vi "ContourPlot v4.6 IV.vi"() -> ()   [LabVIEW 2024]
uses:
  diff para.ctl
  graph para.ctl
  <vilib>/Analysis/NI_AALPro.lvlib
  <vilib>/gmath/NI_Gmath.lvlib
panel:
  out "Field data":dbl[](array[numeric])=[-8.0, -7.95, -7.9, -7.85, -7.8, -7.75, -7.7, -7.65, -7.6, -7.55, -7.5, -7.45, -7.4, -7.35, -7.3, -7.25, -7.2, -7.15, -7.1, -7.05, -7.0, -6.95, -6.9, -6.85, -6.8, -6.75, -6.7, -6.65, -6.6, -6.55, -6.5, -6.45, -6.4, -6.35, -6.3, -6.25, -6.2, -6.15, -6.1, -6.05, -6.0, -5.95, -5.9, -5.85, -5.8, -5.75, -5.7, -5.65, -5.6, -5.55, -5.5, -5.45, -5.4, -5.35, -5.3, -5.25, -5.2, -5.15, -5.1, -5.05, -5.0, -4.95, -4.9, -4.85, -4.8, -4.75, -4.7, -4.65, -4.6, -4.55, -4.5, -4.45, -4.4, -4.35, -4.3, -4.25, -4.2, -4.15, -4.1, -4.05, -4.0, -3.95, -3.9, -3.85, -3.8, -3.75, -3.7, -3.65, -3.6, -3.55, -3.5, -3.45, -3.4, -3.35, -3.3, -3.25, -3.2, -3.15, -3.1, -3.05, -3.0, -2.95, -2.9, -2.85, -2.8, -2.75, -2.7, -2.65, -2.6, -2.55, -2.5, -2.45, -2.4, -2.35, -2.3, -2.25, -2.2, -2.15, -2.1, -2.05, -2.0, -1.95, -1.9, -1.85, -1.8, -1.75, -1.7, -1.65, -1.6, -1.55, -1.5, -1.45, -1.4, -1.35, -1.3, -1.25, -1.2, -1.15, -1.1, -1.05, -1.0, -0.95, -0.9, -0.85, -0.8, -0.75, -0.7, -0.65, -0.6, -0.55, -0.5, -0.45, -0.4, -0.35, -0.3, -0.25, -0.2, -0.15, -0.1, -0.05, 0.0, 0.05, 0.1, 0.15, 0.2, 0.25, 0.3, 0.35, 0.4, 0.45, 0.5, 0.55, 0.6, 0.65, 0.7, 0.75, 0.8, 0.85, 0.9, 0.95, 1.0, 1.05, 1.1, 1.15, 1.2, 1.25, 1.3, 1.35, 1.4, 1.45, 1.5, 1.55, 1.6, 1.65, 1.7, 1.75, 1.8, 1.85, 1.9, 1.95, 2.0, 2.05, 2.1, 2.15, 2.2, 2.25, 2.3, 2.35, 2.4, 2.45, 2.5, 2.55, 2.6, 2.65, 2.7, 2.75, 2.8, 2.85, 2.9, 2.95, 3.0, 3.05, 3.1, 3.15, 3.2, 3.25, 3.3, 3.35, 3.4, 3.45, 3.5, 3.55, 3.6, 3.65, 3.7, 3.75, 3.8, 3.85, 3.9, 3.95, 4.0, 4.05, 4.1, 4.15, 4.2, 4.25, 4.3, 4.35, 4.4, 4.45, 4.5, 4.55, 4.6, 4.65, 4.7, 4.75, 4.8, 4.85, 4.9, 4.95, 5.0, 5.05, 5.1, 5.15, 5.2, 5.25, 5.3, 5.35, 5.4, 5.45, 5.5, 5.55, 5.6, 5.65, 5.7, 5.75, 5.8, 5.85, 5.9, 5.95, 6.0, 6.05, 6.1, 6.15, 6.2, 6.25, 6.3, 6.35, 6.4, 6.45, 6.5, 6.55, 6.6, 6.65, 6.7, 6.75, 6.8, 6.85, 6.9, 6.95, 7.0, 7.05, 7.1, 7.15, 7.2, 7.25, 7.3, 7.35, 7.4, 7.45, 7.5, 7.55, 7.6, 7.65, 7.7, 7.75, 7.8, 7.85, 7.9, 7.95, 8.0]
  in  "Help":bool caption="load data"
  out "smoothed dIV buffer":dbl[][](array[numeric])
  in  "diff para":T1={"x0"=-1.0, "Ic0"=2.0, "h0"=1.0, "y0"=0.0}
  in  "Plot reference":bool caption="load data"
  out "smoothed dIV":dbl[][](array[numeric])
  out "smoothed data":dbl[][](array[numeric])
  in  "smooth n":i32=10
  out "IVdata":dbl[][](array[numeric])
  in  "load data":bool
  out "Status":string="Stopped"
  in  "stop":bool
  in  "Begin":i32
  in  "length":i32=1000
  in  "Contact Resistance":dbl
  in  "Tab Control 2":enum32{"IV plots", "IV smoothed", "dV/dI"}(tab)
  in  "Method":string(combo)="Raw data"
  in  "extract contour":bool caption="load data"
  out "IV Intensity":dbl[][](graph)
  out "IV":T2(graph)
  in  "polynomial order":i32=22
  out "Contour":cluster{"Field data":dbl[], dbl[]}(graph)
  in  "Threshold":dbl
  out "dX/2":dbl=2.3584433814410506
  out "dX":dbl=4.716886762882101
  in  "Plot contour line":bool
  out "IV smoothed intensity":dbl[][](graph)
  out "Smooth IV":cluster{dbl[], "Intensity Graph":dbl[]}(graph)
  in  "Set diff parameter":bool caption="load data"
  out "dVdI Intensity":dbl[][](graph)
  out "dV/dI":cluster{dbl[], "Intensity Graph":dbl[]}(graph)
  in  "book number":i32=820
  in  "file path":path=path "C:/Users/gyue/Desktop/GA01_202401"
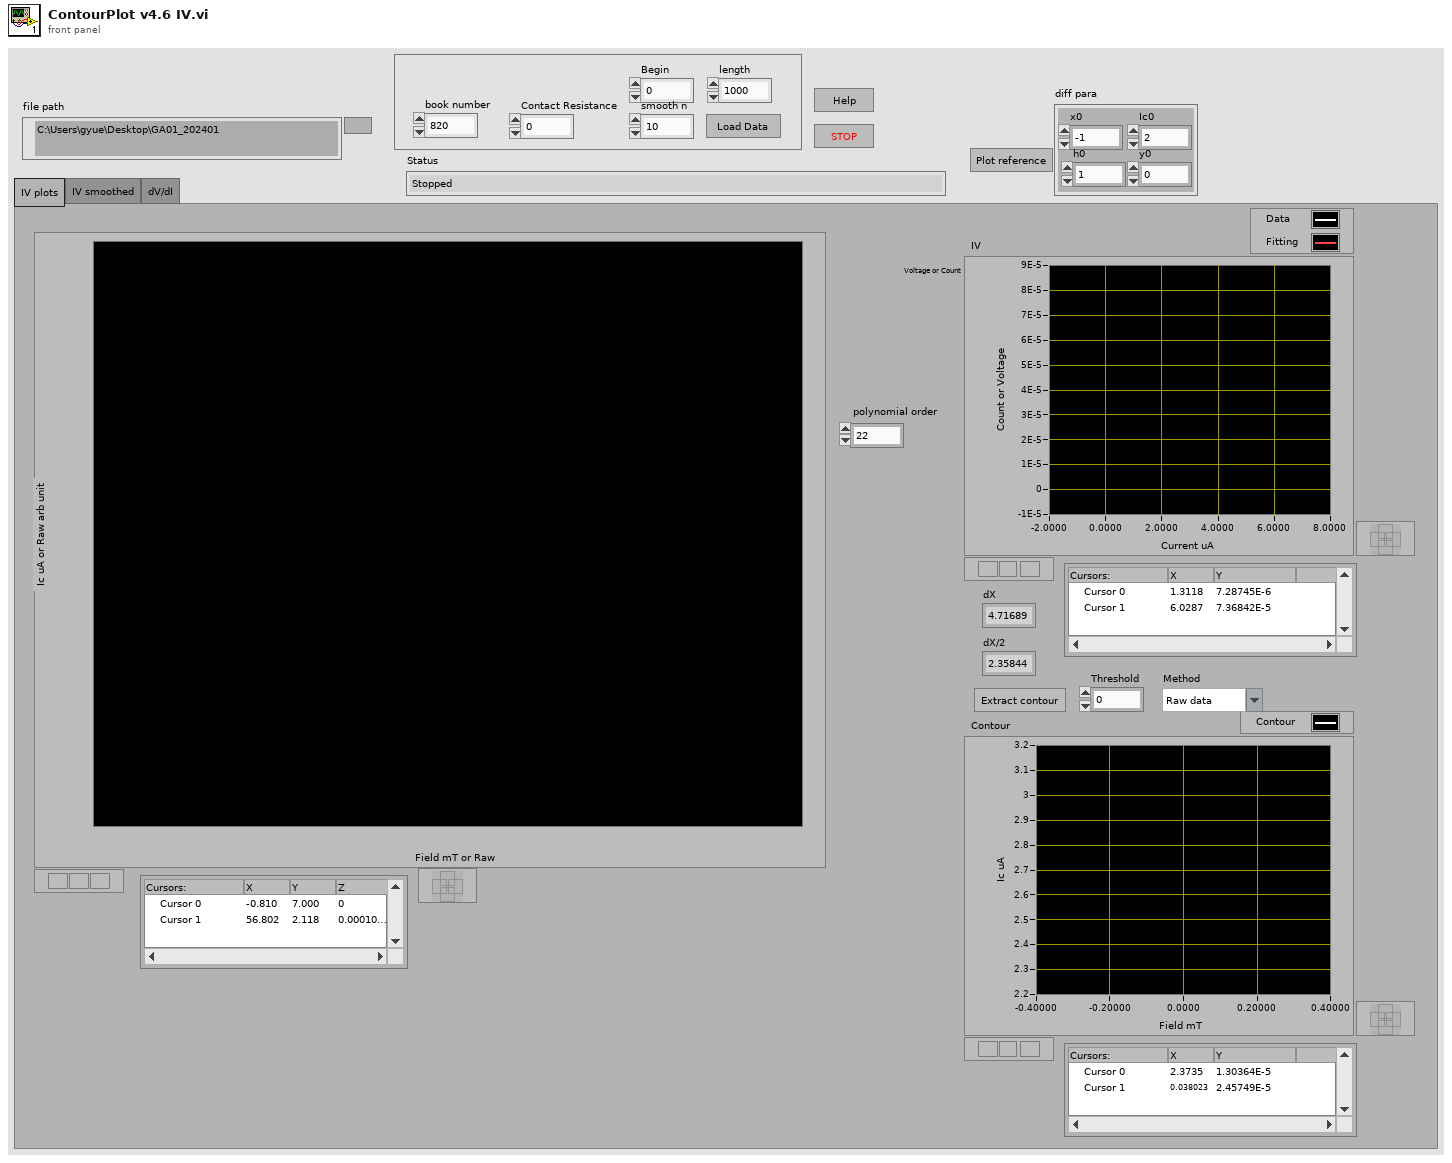
[diagram p1: front panel]
types:
  T1 = typedef "diff para.ctl" = cluster{"x0":dbl, "Ic0":dbl, "h0":dbl, "y0":dbl}
  T2 = cluster{"X":dbl[], "Best Polynomial Fit":dbl[]}[]
  T3 = typedef "graph para.ctl" = cluster{"x offset":dbl, "y offset":dbl, "x scale":dbl, "y scale":dbl}
  T4 = typedef "LVCursorListTypeDef.ctl" = cluster{"Name":string, "Color":u32, "Style":u8, "Point Style":u8, "Name Visible":bool, "Allow Drag":bool, "Cursor Mode":u32, "Plot":i32, "Index":i32, "Position":cluster{"X":dbl, "Y":dbl}, "X Scale":u32, "Y Scale":u32, "Watch Plots":i32[], "Watch All Plots":bool, "Plot Area":i32, "Label Offset":cluster{"X":dbl, "Y":dbl}}[]
  T5 = cluster{"Name":string, "Color":u32, "Style":u8, "Point Style":u8, "Name Visible":bool, "Allow Drag":bool, "Cursor Mode":u32, "Plot":i32, "Index":i32, "Position":cluster{"X":dbl, "Y":dbl}, "X Scale":u32, "Y Scale":u32, "Watch Plots":i32[], "Watch All Plots":bool, "Plot Area":i32, "Label Offset":cluster{"X":dbl, "Y":dbl}}
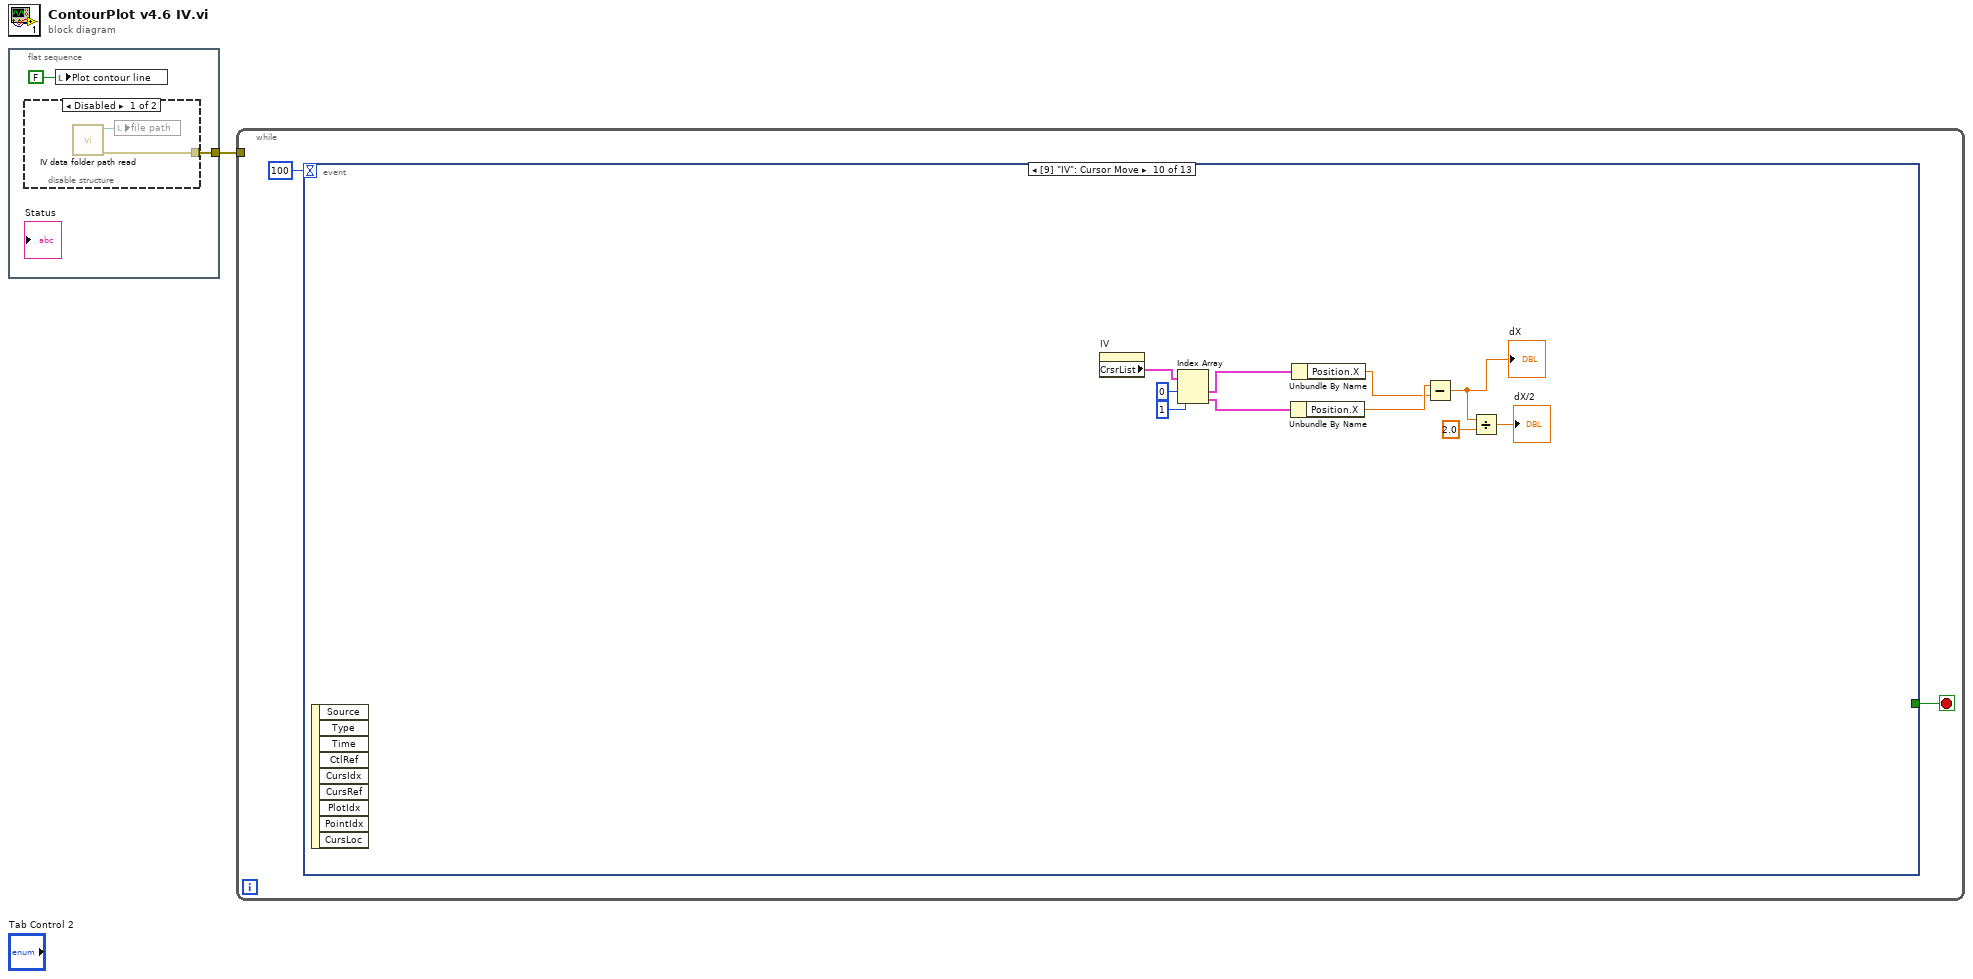
[diagram p0: block diagram]
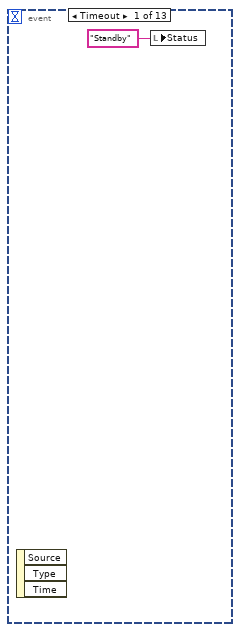
[diagram p3: hidden frame]
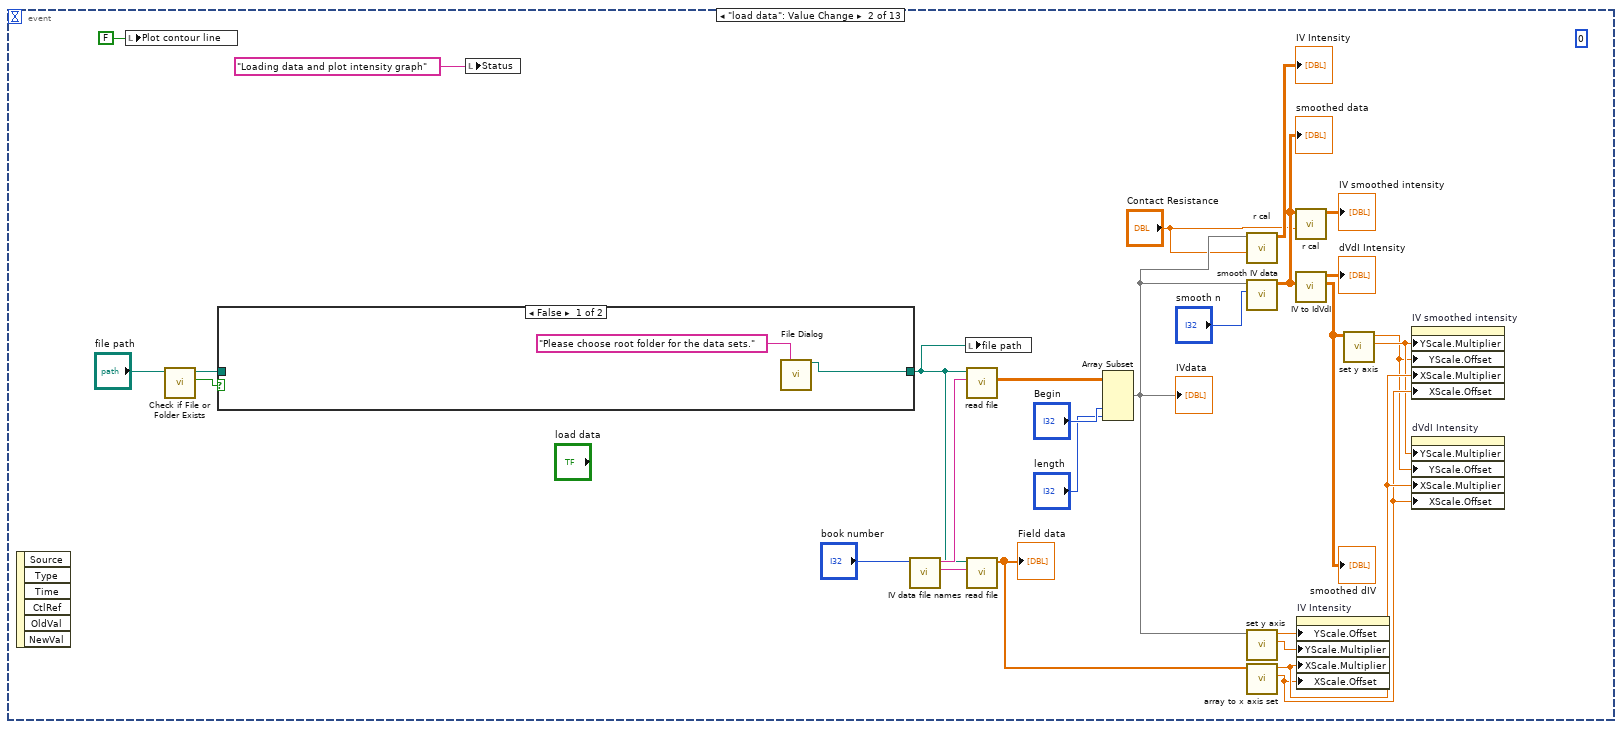
[diagram p4: hidden frame]
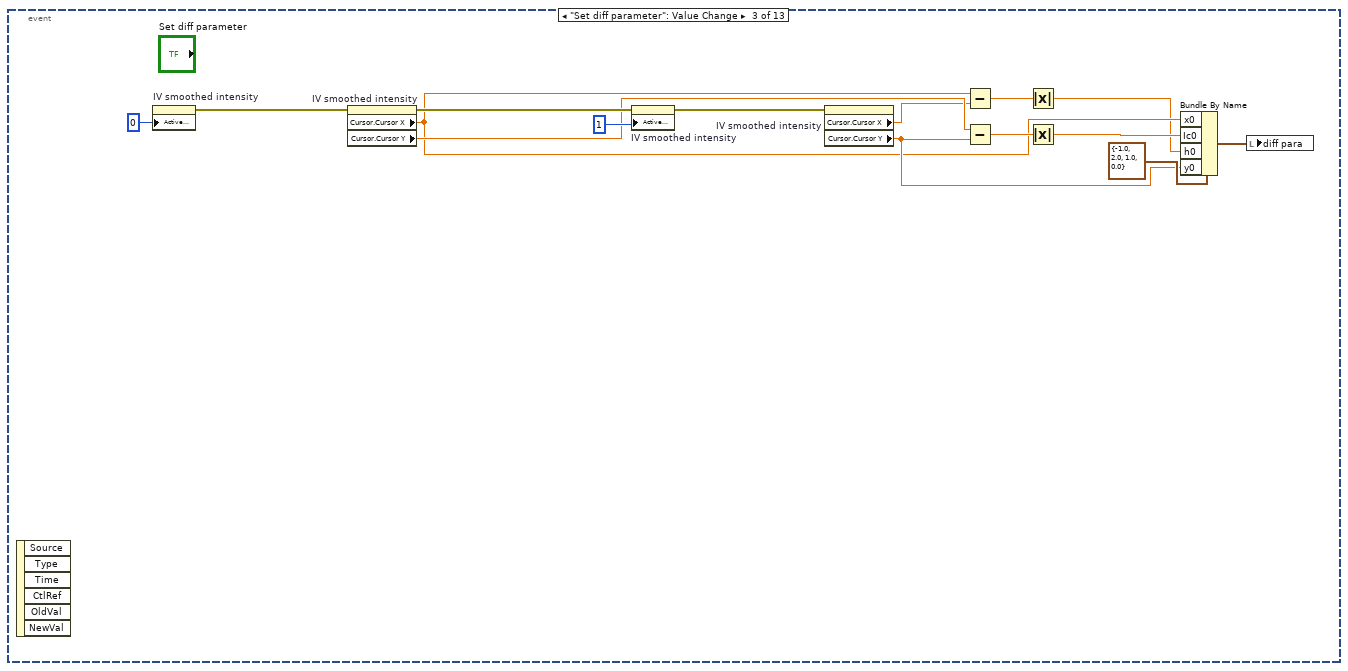
[diagram p6: hidden frame]
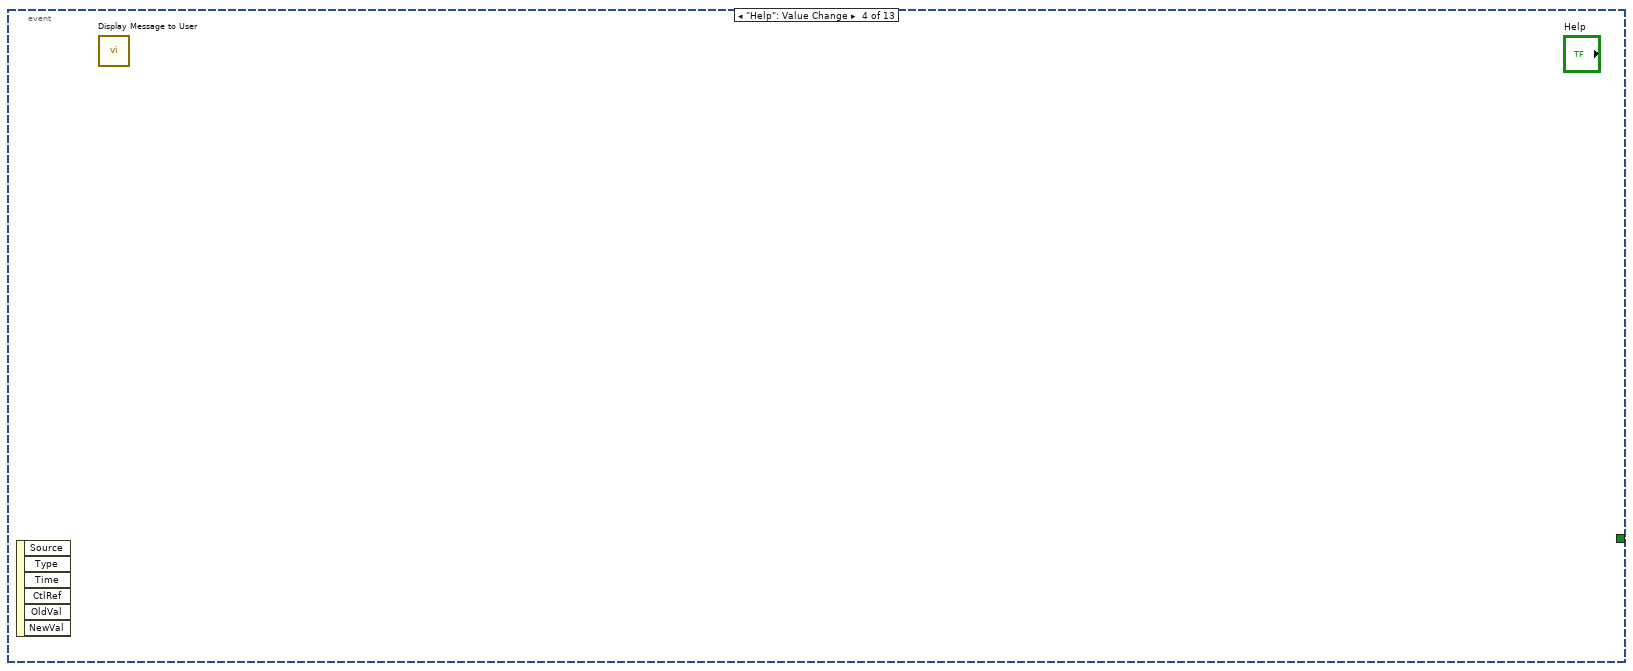
[diagram p7: hidden frame]
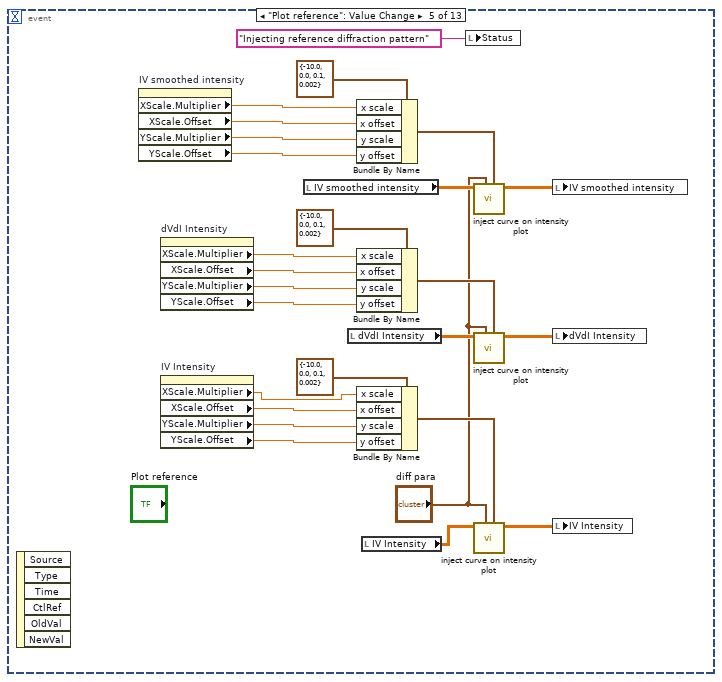
[diagram p8: hidden frame]
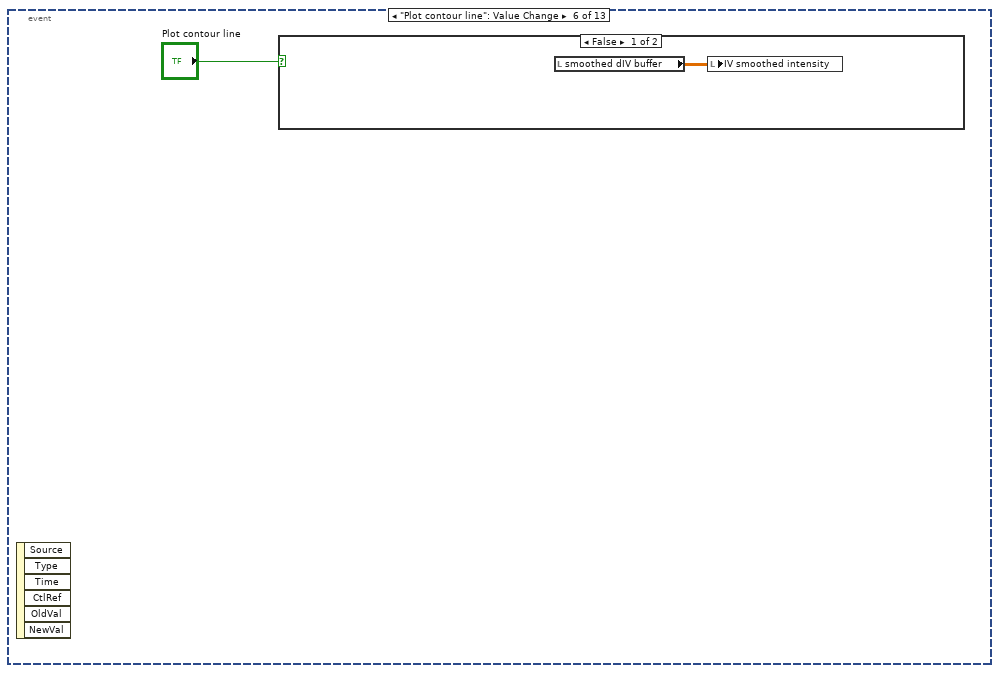
[diagram p9: hidden frame]
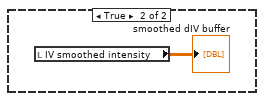
[diagram p10: hidden frame]
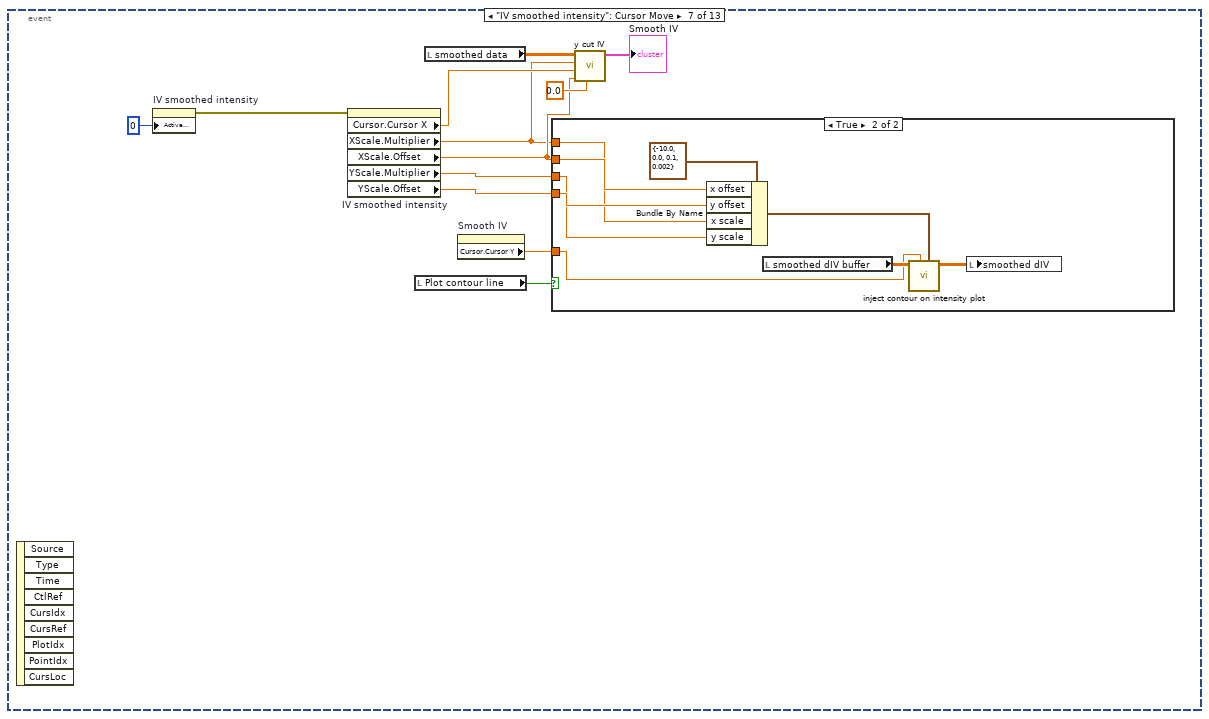
[diagram p11: hidden frame]
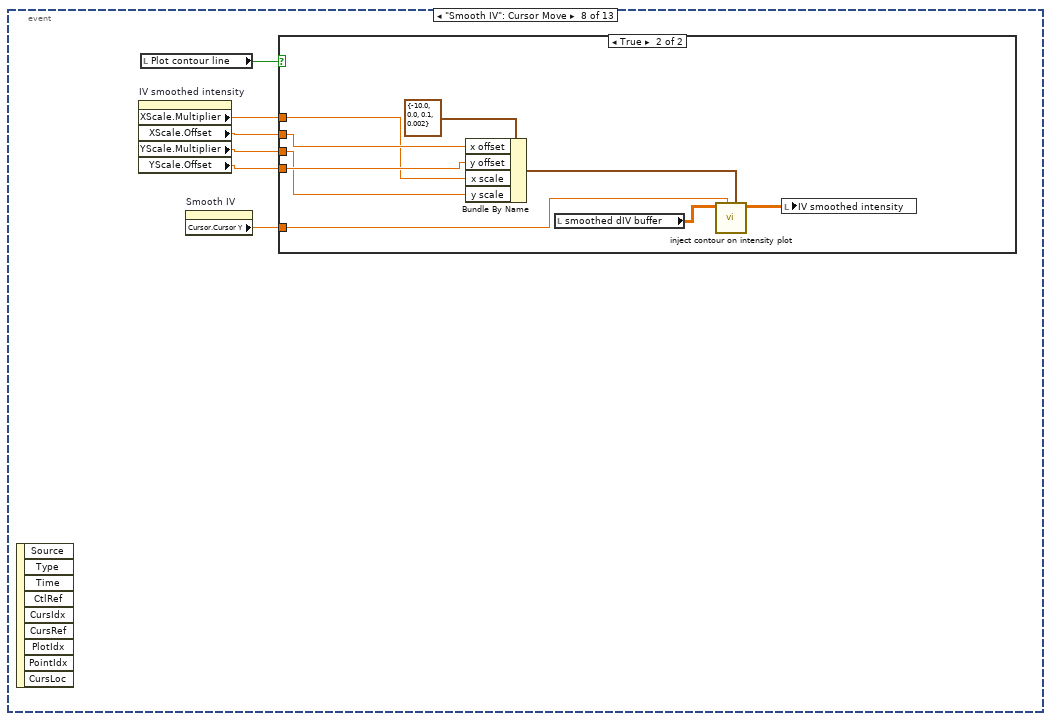
[diagram p13: hidden frame]
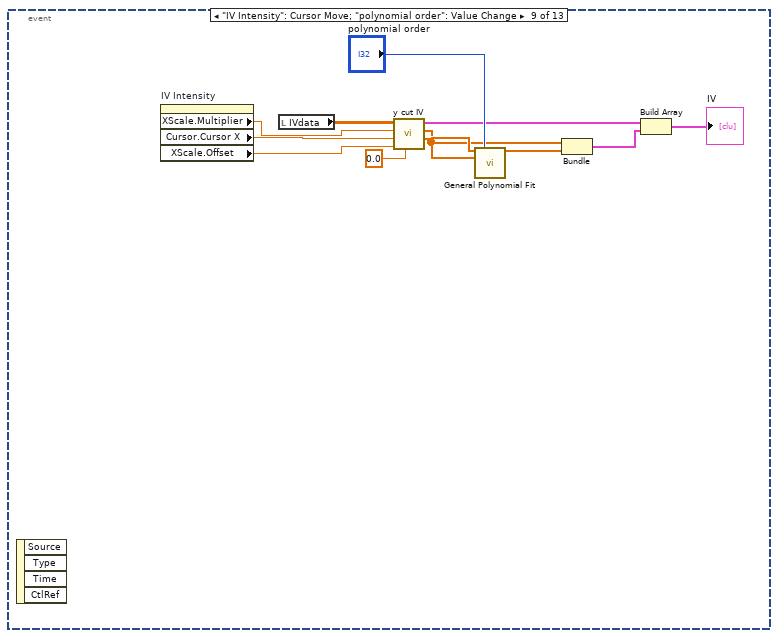
[diagram p15: hidden frame]
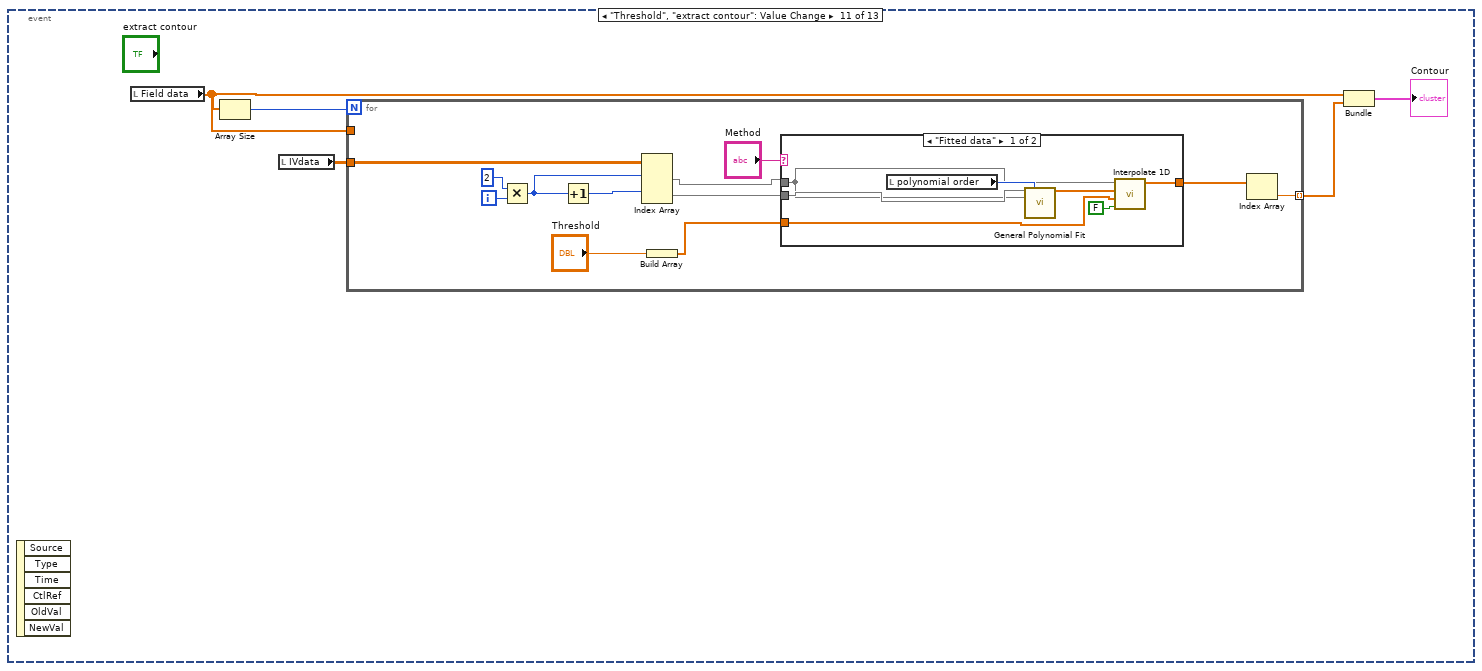
[diagram p16: hidden frame]
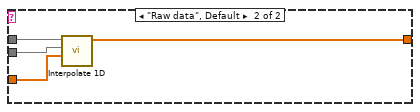
[diagram p17: hidden frame]
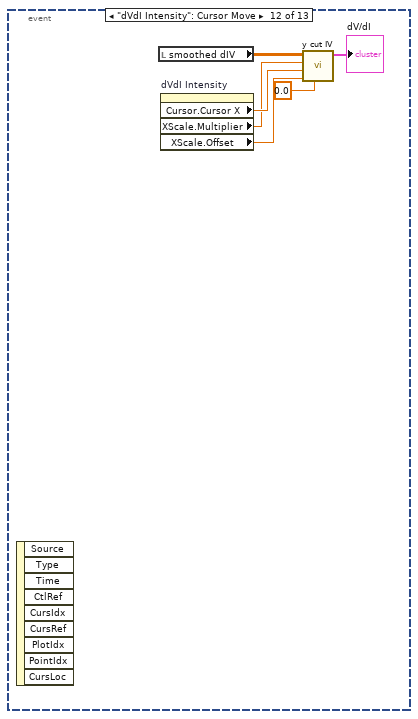
[diagram p18: hidden frame]
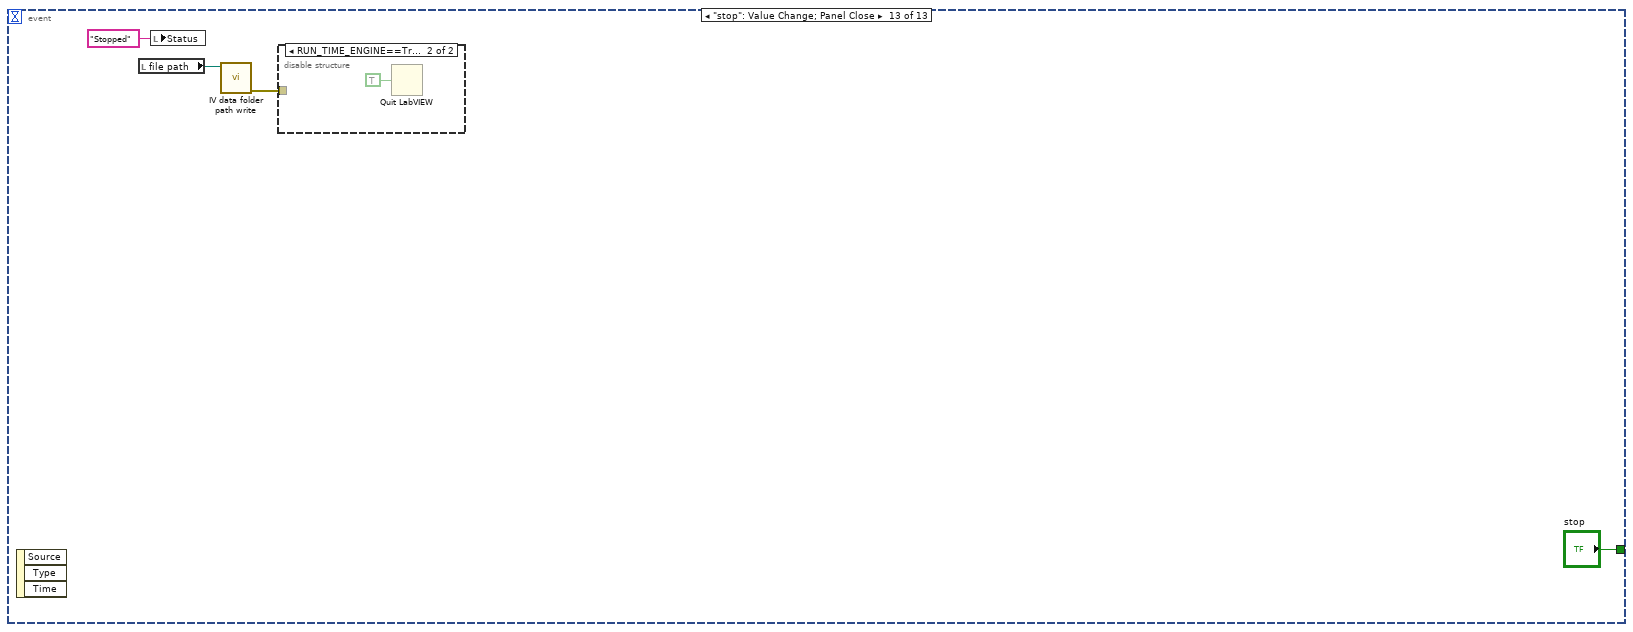
[diagram p19: hidden frame]
diagram:
  n1 = flat-sequence {
    tunnel: [w2] -> w1
    frame #0 {
      n2 = disable-structure shown="Disabled" {
        disable-tunnel: [w4 _] -> w2
        frame Disabled {
          n3 = call "IV data folder path read.vi"() -> ("error out"=w4:errorcluster, "path"=w5:path)  [unwired: 10 in]
          n4 = local write "file path"(w5) -> ()
        }
        frame Enabled {
        }
      }
      n5 = local write "Plot contour line"(FALSE ("Plot contour line")) -> ()
    }
  }
  n6 = while {
    tunnel: w1 -> [_]
    stop <- w6 stop-if-true
    n7 = event shown="[9] \"IV\": Cursor Move" {
      selector: _ -> [_ _ _ _ _ _ _ _ _ _ _ _ _]
      dyn-events: _ -> [_ _ _ _ _ _ _ _ _ _ _ _ _]
      timeout: 100 -> [_ _ _ _ _ _ _ _ _ _ _ _ _]
      tunnel: [_ _ _ _ _ _ _ _ _ _ _ _ "stop"] -> w6
      event Timeout {
        n8 = event-data() -> ()  [unwired: 1 in, 3 out]
        n9 = local write "Status"("Standby" ("Status")) -> ()
      }
      event "load data": Value Change {
        (unwired) 0 ("index (row)")
        n10 = event-data() -> ()  [unwired: 1 in, 6 out]
        n11 = local write "Plot contour line"(FALSE ("Plot contour line")) -> ()
        n12 = call <vilib>:"Check if File or Folder Exists.vi"("path"="file path") -> ("file or folder exists?"=w11:bool, "dup path"=w10:path)  [unwired: 8 in, 1 out]
        n13 = case shown="False" w11 {
          tunnel: [w36 w38] -> w9
          tunnel: w10 -> [_ w38]
          frame False {
            n14 = call "File Dialog"("prompt"="Please choose root folder for the data sets.") -> ("selected path"=w36:path)  [unwired: 11 in, 3 out]
          }
          frame True {
          }
        }
        n15 = local write "Status"("Loading data and plot intensity graph" ("Status")) -> ()
        n16 = call "IV data file names.vi"("book number"="book number") -> ("Field"=w34:string, "IV"=w33:string)  [unwired: 8 in, 1 out]
        n17 = local write "file path"(w9) -> ()
        n18 = call "read file.vi"("file name"=w33, "file path (dialog if empty)"=w9) -> ("2d data"=w26:dbl[][])  [unwired: 8 in, 1 out]
        n19 = call "read file.vi"("file name"=w34, "file path (dialog if empty)"=w9) -> ("1d Data"=w25:dbl[])  [unwired: 8 in, 1 out]
        "Field data" <- w25
        n20 = Array Subset(array=w26, index (col)="Begin", length (col)="length") -> (w22:dbl[][])  [unwired: 2 in]
        "IVdata" <- w22
        n21 = call "r cal.vi"("Contact Resistance"="Contact Resistance", "Array in"=w22) -> ("Array out"=→"IV Intensity":dbl[][])  [unwired: 9 in]
        n22 = call "smooth IV data.vi"("smooth n"="smooth n", "Array in"=w22) -> ("Array out"=w21:dbl[][])  [unwired: 9 in]
        "smoothed data" <- w21
        n23 = call "set y axis.vi"("Array"=w22) -> ("y multi"=w32:dbl, "y offset"=w31:dbl)  [unwired: 9 in]
        n24 = call "array to x axis set.vi"("1d Data"=w25) -> ("offset"=w17:dbl, "multiplier"=w18:dbl)  [unwired: 9 in]
        n25 = call "r cal.vi"("Contact Resistance"="Contact Resistance", "Array in"=w21) -> ("Array out"=→"IV smoothed intensity":dbl[][])  [unwired: 9 in]
        n26 = call "IV to IdVdI.vi"("Array in"=w21) -> ("Array"=w16:dbl[][], "Array 2"=→"dVdI Intensity":dbl[][])  [unwired: 9 in]
        "smoothed dIV" <- w16
        n27 = property on="IV Intensity" class="IntGraph (strict)"("YScale.Offset"=w31, "YScale.Multiplier"=w32, "XScale.Multiplier"=w18, "XScale.Offset"=w17) -> ()  [unwired: 2 in, 2 out]
        n28 = call "set y axis.vi"("Array"=w16) -> ("y multi"=w15:dbl, "y offset"=w14:dbl)  [unwired: 9 in]
        n29 = property on="IV smoothed intensity" class="IntGraph (strict)"("YScale.Multiplier"=w15, "YScale.Offset"=w14, "XScale.Multiplier"=w18, "XScale.Offset"=w17) -> ()  [unwired: 2 in, 2 out]
        n30 = property on="dVdI Intensity" class="IntGraph (strict)"("YScale.Multiplier"=w15, "YScale.Offset"=w14, "XScale.Multiplier"=w18, "XScale.Offset"=w17) -> ()  [unwired: 2 in, 2 out]
      }
      event "Set diff parameter": Value Change {
        n31 = event-data() -> ()  [unwired: 1 in, 6 out]
        n32 = property on="IV smoothed intensity" class="IntGraph (strict)"("Active Cursor"=u32 0) -> (error out=w53:errorcluster)  [unwired: 2 in, 1 out]
        n33 = property on="IV smoothed intensity" class="IntGraph (strict)"(error in=w53) -> (error out=w50:errorcluster, "Cursor.Cursor X"=w42:dbl, "Cursor.Cursor Y"=w46:dbl)  [unwired: 1 in, 1 out]
        n34 = property on="IV smoothed intensity" class="IntGraph (strict)"(error in=w50, "Active Cursor"=u32 1) -> (error out=w49:errorcluster)  [unwired: 1 in, 1 out]
        n35 = property on="IV smoothed intensity" class="IntGraph (strict)"(error in=w49) -> ("Cursor.Cursor X"=w41:dbl, "Cursor.Cursor Y"=w45:dbl)  [unwired: 1 in, 2 out]
        n36 = Subtract(x=w42, y=w41) -> (x-y=w40:dbl)
        n37 = Subtract(x=w46, y=w45) -> (x-y=w44:dbl)
        n38 = Absolute Value(x=w40) -> (abs(x)=w39:dbl)
        n39 = Absolute Value(x=w44) -> (abs(x)=w43:dbl)
        n40 = Bundle By Name(cluster=T1 {"x0"=-1.0, "Ic0"=2.0, "h0"=1.0, "y0"=0.0} ("diff para"), "x0"=w42, "Ic0"=w43, "h0"=w39, "y0"=w45) -> (w48:T1)
        n41 = local write "diff para"(w48) -> ()
      }
      event "Help": Value Change {
        n42 = event-data() -> ()  [unwired: 1 in, 6 out]
        n43 = call "Display Message to User"() -> ()  [unwired: 10 in, 2 out]
      }
      event "Plot reference": Value Change {
        n44 = event-data() -> ()  [unwired: 1 in, 6 out]
        n45 = property on="IV smoothed intensity" class="IntGraph (strict)"() -> ("XScale.Multiplier"=w65:dbl, "XScale.Offset"=w64:dbl, "YScale.Multiplier"=w63:dbl, "YScale.Offset"=w62:dbl)  [unwired: 2 in, 2 out]
        n46 = property on="dVdI Intensity" class="IntGraph (strict)"() -> ("XScale.Multiplier"=w59:dbl, "XScale.Offset"=w58:dbl, "YScale.Multiplier"=w57:dbl, "YScale.Offset"=w56:dbl)  [unwired: 2 in, 2 out]
        n47 = property on="IV Intensity" class="IntGraph (strict)"() -> ("XScale.Multiplier"=w77:dbl, "XScale.Offset"=w76:dbl, "YScale.Multiplier"=w75:dbl, "YScale.Offset"=w74:dbl)  [unwired: 2 in, 2 out]
        n48 = local read "IV smoothed intensity"() -> (w66:dbl[][])
        n49 = local read "dVdI Intensity"() -> (w60:dbl[][])
        n50 = Bundle By Name(cluster=T3 {"x offset"=-10.0, "y offset"=0.0, "x scale"=0.1, "y scale"=0.002} ("graph para"), "x scale"=w65, "x offset"=w64, "y scale"=w63, "y offset"=w62) -> (w69:T3)
        n51 = Bundle By Name(cluster=T3 {"x offset"=-10.0, "y offset"=0.0, "x scale"=0.1, "y scale"=0.002} ("graph para"), "x scale"=w59, "x offset"=w58, "y scale"=w57, "y offset"=w56) -> (w67:T3)
        n52 = Bundle By Name(cluster=T3 {"x offset"=-10.0, "y offset"=0.0, "x scale"=0.1, "y scale"=0.002} ("graph para"), "x scale"=w77, "x offset"=w76, "y scale"=w75, "y offset"=w74) -> (w73:T3)
        n53 = local read "IV Intensity"() -> (w79:dbl[][])
        n54 = local write "Status"("Injecting reference diffraction pattern" ("Status")) -> ()
        n55 = call "inject curve on intensity plot.vi"("graph para"=w69, "diff para"="diff para", "IV Intensity"=w66) -> ("IV Intensity 2"=w61:dbl[][])  [unwired: 8 in]
        n56 = call "inject curve on intensity plot.vi"("graph para"=w67, "diff para"="diff para", "IV Intensity"=w60) -> ("IV Intensity 2"=w54:dbl[][])  [unwired: 8 in]
        n57 = call "inject curve on intensity plot.vi"("graph para"=w73, "diff para"="diff para", "IV Intensity"=w79) -> ("IV Intensity 2"=w72:dbl[][])  [unwired: 8 in]
        n58 = local write "IV smoothed intensity"(w61) -> ()
        n59 = local write "dVdI Intensity"(w54) -> ()
        n60 = local write "IV Intensity"(w72) -> ()
      }
      event "Plot contour line": Value Change {
        n61 = event-data() -> ()  [unwired: 1 in, 6 out]
        n62 = case shown="False" "Plot contour line" {
          frame False {
            n63 = local read "smoothed dIV buffer"() -> (w81:dbl[][])
            n64 = local write "IV smoothed intensity"(w81) -> ()
          }
          frame True {
            n65 = local read "IV smoothed intensity"() -> (→"smoothed dIV buffer":dbl[][])
          }
        }
      }
      event "IV smoothed intensity": Cursor Move {
        n66 = event-data() -> ()  [unwired: 1 in, 9 out]
        n67 = property on="IV smoothed intensity" class="IntGraph (strict)"("Active Cursor"=u32 0) -> (error out=w83:errorcluster)  [unwired: 2 in, 1 out]
        n68 = property on="IV smoothed intensity" class="IntGraph (strict)"(error in=w83) -> ("Cursor.Cursor X"=w91:dbl, "XScale.Multiplier"=w87:dbl, "XScale.Offset"=w89:dbl, "YScale.Multiplier"=w86:dbl, "YScale.Offset"=w88:dbl)  [unwired: 1 in, 2 out]
        n69 = local read "Plot contour line"() -> (w90:bool)
        n70 = local read "smoothed data"() -> (w94:dbl[][])
        n71 = property on="Smooth IV" class="XYGraph (strict)"() -> ("Cursor.Cursor Y"=w85:dbl)  [unwired: 2 in, 2 out]
        n72 = case shown="True" w90 {
          tunnel: w85 -> [_ w101]
          tunnel: w89 -> [_ w99]
          tunnel: w88 -> [_ w98]
          tunnel: w87 -> [_ w97]
          tunnel: w86 -> [_ w96]
          frame False {
          }
          frame True {
            n73 = Bundle By Name(cluster=T3 {"x offset"=-10.0, "y offset"=0.0, "x scale"=0.1, "y scale"=0.002} ("graph para"), "x offset"=w99, "y offset"=w98, "x scale"=w97, "y scale"=w96) -> (w95:T3)
            n74 = local read "smoothed dIV buffer"() -> (w103:dbl[][])
            n75 = call "inject contour on intensity plot.vi"("graph para"=w95, "Threshold"=w101, "IV Intensity"=w103) -> ("IV Intensity output"=w102:dbl[][])  [unwired: 6 in, 2 out]
            n76 = local write "smoothed dIV"(w102) -> ()
          }
        }
        n77 = call "y cut IV.vi"("Contact Resistance"=0.0, "x offset"=w89, "x pos"=w91, "scale"=w87, "Data"=w94) -> ("IV"=→"Smooth IV":cluster{"Data":dbl[], dbl[]})  [unwired: 4 in, 2 out]
      }
      event "Smooth IV": Cursor Move {
        n78 = event-data() -> ()  [unwired: 1 in, 9 out]
        n79 = property on="IV smoothed intensity" class="IntGraph (strict)"() -> ("XScale.Multiplier"=w106:dbl, "XScale.Offset"=w108:dbl, "YScale.Multiplier"=w105:dbl, "YScale.Offset"=w107:dbl)  [unwired: 2 in, 2 out]
        n80 = local read "Plot contour line"() -> (w109:bool)
        n81 = property on="Smooth IV" class="XYGraph (strict)"() -> ("Cursor.Cursor Y"=w104:dbl)  [unwired: 2 in, 2 out]
        n82 = case shown="True" w109 {
          tunnel: w104 -> [_ w116]
          tunnel: w108 -> [_ w114]
          tunnel: w107 -> [_ w113]
          tunnel: w106 -> [_ w112]
          tunnel: w105 -> [_ w111]
          frame False {
          }
          frame True {
            n83 = Bundle By Name(cluster=T3 {"x offset"=-10.0, "y offset"=0.0, "x scale"=0.1, "y scale"=0.002} ("graph para"), "x offset"=w114, "y offset"=w113, "x scale"=w112, "y scale"=w111) -> (w110:T3)
            n84 = local read "smoothed dIV buffer"() -> (w118:dbl[][])
            n85 = call "inject contour on intensity plot.vi"("graph para"=w110, "Threshold"=w116, "IV Intensity"=w118) -> ("IV Intensity output"=w117:dbl[][])  [unwired: 6 in, 2 out]
            n86 = local write "IV smoothed intensity"(w117) -> ()
          }
        }
      }
      event "IV Intensity": Cursor Move; "polynomial order": Value Change {
        n87 = event-data() -> ()  [unwired: 1 in, 4 out]
        n88 = property on="IV Intensity" class="IntGraph (strict)"() -> ("XScale.Multiplier"=w128:dbl, "Cursor.Cursor X"=w129:dbl, "XScale.Offset"=w130:dbl)  [unwired: 2 in, 2 out]
        n89 = local read "IVdata"() -> (w127:dbl[][])
        n90 = call "y cut IV.vi"("Contact Resistance"=0.0, "x offset"=w130, "x pos"=w129, "scale"=w128, "Data"=w127) -> ("Y"=w124:dbl[], "X"=w122:dbl[], "IV"=w123:cluster{"Data":dbl[], dbl[]})  [unwired: 4 in]
        n91 = call <vilib>:"General Polynomial Fit.vi"("Y"=w124, "polynomial order"="polynomial order", "X"=w122) -> ("Best Polynomial Fit"=w121:dbl[])  [unwired: 9 in, 3 out]
        n92 = Bundle("X"=w122, "Best Polynomial Fit"=w121) -> (w120:cluster{"X":dbl[], "Best Polynomial Fit":dbl[]})  [unwired: 1 in]
        n93 = Build Array(w123, w120) -> (→"IV":T2)
      }
      event "IV": Cursor Move {
        n94 = event-data() -> ()  [unwired: 1 in, 9 out]
        n95 = property on="IV" class="XYGraph (strict)"() -> ("CrsrList"=w140:T4)  [unwired: 2 in, 2 out]
        n96 = Index Array(array=w140, index #1=0 ("index"), index #2=1 ("index")) -> (element #1=w137:T5, element #2=w136:T5)
        n97 = Unbundle By Name(w136) -> ("Position.X"=w135:dbl)
        n98 = Unbundle By Name(w137) -> ("Position.X"=w134:dbl)
        n99 = Subtract(x=w135, y=w134) -> (x-y=w133:dbl)
        "dX" <- w133
        n100 = Divide(x=w133, y=2.0) -> (x/y=→"dX/2":dbl)
      }
      event "Threshold", "extract contour": Value Change {
        n101 = event-data() -> ()  [unwired: 1 in, 6 out]
        n102 = local read "Field data"() -> (w142:dbl[])
        n103 = Array Size(array=w142) -> (size(s)=w141:i32)
        n104 = local read "IVdata"() -> (w144:dbl[][])
        n105 = for {
          N: w141 -> [_]
          tunnel: w142 -> [_]
          tunnel: w144 -> [w155]
          tunnel: [w147] -> w143 mode=indexing
          i -> [w157]
          n106 = Multiply(x=2, y=w157) -> (x*y=w154:i32)
          n107 = Increment(x=w154) -> (x+1=w153:i32)
          n108 = Index Array(array=w155, index (row) #1=w154, index (row) #2=w153) -> (element #1=w152:dbl[], element #2=w151:dbl[])  [unwired: 2 in]
          n109 = Build Array("Threshold") -> (w149:dbl[])
          n110 = case shown="\"Fitted data\"" "Method" {
            tunnel: w152 -> [w162 w168]
            tunnel: w151 -> [w164 w167]
            tunnel: w149 -> [w160 w166]
            tunnel: [w158 w165] -> w148
            frame "Fitted data" {
              n111 = local read "polynomial order"() -> (w163:i32)
              n112 = call <vilib>:"General Polynomial Fit.vi"("Y"=w164, "polynomial order"=w163, "X"=w162) -> ("Best Polynomial Fit"=w161:dbl[])  [unwired: 9 in, 3 out]
              n113 = call <vilib>:"Interpolate 1D.vi"("X is monotonic"=FALSE, "xi"=w160, "X"=w161, "Y"=w162) -> ("yi"=w158:dbl[])  [unwired: 5 in, 2 out]
            }
            frame "Raw data", Default {
              n114 = call <vilib>:"Interpolate 1D.vi"("xi"=w166, "X"=w167, "Y"=w168) -> ("yi"=w165:dbl[])  [unwired: 6 in, 2 out]
            }
          }
          n115 = Index Array(array=w148) -> (element=w147:dbl)  [unwired: 1 in]
        }
        n116 = Bundle("Field data"=w142, w143) -> (→"Contour":cluster{"Field data":dbl[], dbl[]})  [unwired: 1 in]
      }
      event "dVdI Intensity": Cursor Move {
        n117 = event-data() -> ()  [unwired: 1 in, 9 out]
        n118 = local read "smoothed dIV"() -> (w174:dbl[][])
        n119 = property on="dVdI Intensity" class="IntGraph (strict)"() -> ("Cursor.Cursor X"=w172:dbl, "XScale.Multiplier"=w171:dbl, "XScale.Offset"=w170:dbl)  [unwired: 2 in, 2 out]
        n120 = call "y cut IV.vi"("Contact Resistance"=0.0, "x offset"=w170, "x pos"=w172, "scale"=w171, "Data"=w174) -> ("IV"=→"dV/dI":cluster{"Data":dbl[], dbl[]})  [unwired: 4 in, 2 out]
      }
      event "stop": Value Change; Panel Close {
        n121 = event-data() -> ()  [unwired: 1 in, 3 out]
        n122 = local read "file path"() -> (w176:path)
        n123 = local write "Status"("Stopped" ("Status")) -> ()
        n124 = call "IV data folder path write.vi"("Path"=w176) -> ("error out"=w175:errorcluster)  [unwired: 10 in]
        n125 = disable-structure shown="RUN_TIME_ENGINE==True" {
          disable-tunnel: w175 -> [_ _]
          frame condition #0 (active) {
          }
          frame condition #1 {
            n126 = Quit LabVIEW(quit? (T)=TRUE) -> ()
          }
        }
      }
    }
  }
